vi "HFRR ADV v043.vi"() -> ()   [LabVIEW 2025] (continued)
      tunnel: [FALSE FALSE FALSE _ FALSE _ _ _ _ _ _ _ _ _ _ _ _ _ _ _ _ _ _ _ _ _ _ _ _ _ _ _ _ _ _ _ _ _ _ _ _ _ _ _ _ _ _ _ _ _ _ _ _ _ _ _ TRUE] -> w383
      event Timeout {
        n287 = event-data() -> ()  [unwired: 1 in, 3 out]
        n288 = disable-structure shown="Disabled" {
          frame Disabled {
            n289 = local read "Auto Start Test"() -> (w397:bool)
            n290 = local read "RUN"() -> (w398:bool)
            n291 = Or(x=w398, y=w397) -> (x .or. y?=w396:bool)
            n292 = case shown="True" w396 {
              frame False {
                w399 = TRUE ("PAUSE")
                n293 = call "ELAPSED TIMER VI - abort test.vi"("RESET"=w399, "PAUSE"=w399) -> ()  [unwired: 7 in, 3 out]
              }
              frame True {
                n294 = local read "Stroke 2"() -> (w404:dbl)
                n295 = local read "FF 3"() -> (w406:dbl)
                n296 = Equal?(x=w404, y=0.95 ("Stroke 2")) -> (x = y?=w401:bool)
                n297 = Equal?(x=w406, y=0.0 ("FF 3")) -> (x = y?=w402:bool)
                n298 = Or(x=w402, y=w401) -> (x .or. y?=w400:bool)
                n299 = case shown="True" w400 {
                  selector: w400 -> [_ w411]
                  frame False {
                    w407 = TRUE ("PAUSE")
                    n300 = call "ELAPSED TIMER VI - abort test.vi"("RESET"=w407, "PAUSE"=w407) -> ()  [unwired: 7 in, 3 out]
                  }
                  frame True {
                    n301 = Not(x=w411) -> (.not. x?=w410:bool)
                    n302 = call "ELAPSED TIMER VI - abort test.vi"("TARGET"=60.0, "RESET"=w410, "PAUSE"=FALSE) -> ("ELAPSED INDICATION"=w408:bool)  [unwired: 6 in, 2 out]
                    n303 = case shown="True" w408 {
                      frame False {
                      }
                      frame True {
                        n304 = stacked-sequence {
                          frame #0 {
                            w413 = FALSE
                            n305 = local write "RUN"(w413) -> ()
                            n306 = local write "Auto Start Test"(w413) -> ()
                          }
                          frame #1 {
                            n307 = One Button Dialog(message="Test stopped due to a communication error. Reconnect the C1 and C2 cables.") -> ()  [unwired: 1 in, 1 out]
                          }
                        }
                      }
                    }
                  }
                }
              }
            }
          }
          frame Enabled {
          }
        }
        n308 = Get Date/Time In Seconds() -> (seconds since 1Jan1904=w394:timestamp)
        n309 = Format Into String(format string="%<%I:%M:%S:%p %d:%B:%Y>T", w394) -> (resulting string=→"Time Stamp":string)  [unwired: 2 in, 1 out]
        n310 = local read "Service Password enable"() -> (w386:bool)
        n311 = local read "FILE"() -> (w391:string)
        n312 = call <vilib>:"Trim Whitespace.vi"("string"=w391) -> ("trimmed string"=w390:string)  [unwired: 1 in]
        n313 = String Length(string=w390) -> (length=w389:i32)
        n314 = Greater?(x=w389, y=1) -> (0:w387:bool)
        n315 = case shown="False" w387 {
          tunnel: w386 -> [w415 _]
          frame False {
            n316 = case shown="False" w415 {
              frame True {
                w416 = "Test Start In Service Mode" ("Tip Strip")
                w417 = T19."Enabled" ("Disabled")
                n317 = property on="Auto Start Test" class="Bool (strict)"("DisabledEnum"=w417, "TipStrip"=w416) -> ()  [unwired: 2 in, 2 out]
                n318 = property on="RUN" class="Bool (strict)"("DisabledEnum"=w417, "TipStrip"=w416) -> ()  [unwired: 2 in, 2 out]
              }
              frame False {
                w418 = "Enter File Name to Start Test" ("Tip Strip")
                w419 = T19."Disabled and Grayed Out" ("Disabled")
                n319 = property on="Auto Start Test" class="Bool (strict)"("DisabledEnum"=w419, "TipStrip"=w418) -> ()  [unwired: 2 in, 2 out]
                n320 = property on="RUN" class="Bool (strict)"("DisabledEnum"=w419, "TipStrip"=w418) -> ()  [unwired: 2 in, 2 out]
              }
            }
          }
          frame True {
            w420 = "" ("Tip Strip")
            w421 = T19."Enabled" ("Disabled")
            n321 = property on="Auto Start Test" class="Bool (strict)"("DisabledEnum"=w421, "TipStrip"=w420) -> ()  [unwired: 2 in, 2 out]
            n322 = property on="RUN" class="Bool (strict)"("DisabledEnum"=w421, "TipStrip"=w420) -> ()  [unwired: 2 in, 2 out]
          }
        }
      }
      event "RUN": Value Change {
        n323 = event-data() -> ()  [unwired: 1 in, 6 out]
        n324 = local read "RUN"() -> (w423:bool)
        n325 = case shown="False" w423 {
          frame False {
            n326 = flat-sequence {
              frame #0 {
                n327 = local write "START TEMP"(FALSE ("START TEMP")) -> ()
              }
              frame #1 {
                n328 = Wait (ms)(milliseconds to wait=u32 1500) -> ()  [unwired: 1 out]
              }
              frame #2 {
                n329 = local write "Humidity 2"(TRUE ("Humidity")) -> ()
              }
              frame #3 {
                n330 = local write "Due Write"("VC;0") -> ()
              }
              frame #4 {
                n331 = Wait (ms)(milliseconds to wait=u32 1500) -> ()  [unwired: 1 out]
              }
              frame #5 {
                w433 = T19."Enabled" ("Disabled")
                (unwired) T25."Imaging" ("Main Dashboard Buttons")
                (unwired) T21."Adv Scar" ("Main Tab")
                w435 = "" ("FILE")
                n332 = local write "measured_stroke"(0.0 ("measured_stroke")) -> ()
                n333 = local write "Due Write"("VC;0") -> ()
                n334 = local write "FILE"(w435) -> ()
                n335 = local write "Batch Ref Num :"(w435) -> ()
                n336 = local write "Fuel Discription :"(w435) -> ()
                n337 = local write "Main Tab"(T2."Adv Scar" ("Main Tab")) -> ()
                n338 = local write "Remarks :"(w435) -> ()
                n339 = local write "Main Dashboard Buttons"(T1."Imaging" ("Main Dashboard Buttons")) -> ()
                n340 = local write "TEST FILE NAM,E SAVED"(FALSE ("TEST FILE NAM,E SAVED")) -> ()
                n341 = property on="Stroke ( mm )" class="WFChart (strict)"("History Data"=cluster{"y":dbl, dbl, "y":dbl}[] []) -> ()  [unwired: 2 in, 2 out]
                n342 = property on="Auto Start Test" class="Bool (strict)"("Visible"=TRUE) -> ()  [unwired: 2 in, 2 out]
                n343 = property on="FRICVALZ 2" class="Bool (strict)"("DisabledEnum"=w433) -> ()  [unwired: 2 in, 2 out]
                n344 = property on="FRICVALZ 4" class="Bool (strict)"("DisabledEnum"=w433) -> ()  [unwired: 2 in, 2 out]
                n345 = property on="FRICVALZ 3" class="Bool (strict)"("DisabledEnum"=w433) -> ()  [unwired: 2 in, 2 out]
              }
            }
          }
          frame True {
            n346 = stacked-sequence {
              frame #0 {
                n347 = local write "FRICVALZ 4"(TRUE ("FRICVALZ 4")) -> ()
                n348 = local write "Due Write"("DAC;200") -> ()
              }
              frame #1 {
              }
              frame #2 {
              }
              frame #3 {
                n349 = Wait (ms)(milliseconds to wait=u32 1000) -> ()  [unwired: 1 out]
              }
              frame #4 {
                n350 = local write "Due Write"("VC;1") -> ()
              }
              frame #5 {
                n351 = Wait (ms)(milliseconds to wait=u32 1000) -> ()  [unwired: 1 out]
              }
              frame #6 {
                n352 = local write "Due Write"("VC;1") -> ()
              }
              frame #7 {
                n353 = Wait (ms)(milliseconds to wait=u32 1500) -> ()  [unwired: 1 out]
              }
              frame #8 {
                w446 = T19."Disabled" ("Disabled")
                n354 = property on="Auto Start Test" class="Bool (strict)"("Visible"=FALSE) -> ()  [unwired: 2 in, 2 out]
                n355 = local write "START TEMP"(TRUE ("START TEMP")) -> ()
                n356 = property on="FRICVALZ 2" class="Bool (strict)"("DisabledEnum"=w446) -> ()  [unwired: 2 in, 2 out]
                n357 = property on="FRICVALZ 4" class="Bool (strict)"("DisabledEnum"=w446) -> ()  [unwired: 2 in, 2 out]
                n358 = property on="FRICVALZ 3" class="Bool (strict)"("DisabledEnum"=w446) -> ()  [unwired: 2 in, 2 out]
              }
            }
          }
        }
      }
      event "run test Calibration": Value Change {
        n359 = event-data() -> ()  [unwired: 1 in, 6 out]
        n360 = local read "run test Calibration"() -> (w448:bool)
        n361 = case shown="False" w448 {
          frame False {
            n362 = flat-sequence {
              frame #0 {
                n363 = local write "START TEMP"(FALSE ("START TEMP")) -> ()
              }
              frame #1 {
                n364 = Wait (ms)(milliseconds to wait=u32 1500) -> ()  [unwired: 1 out]
              }
              frame #2 {
              }
              frame #3 {
                n365 = local write "Due Write"("VC;0") -> ()
              }
              frame #4 {
                n366 = Wait (ms)(milliseconds to wait=u32 1500) -> ()  [unwired: 1 out]
              }
              frame #5 {
                n367 = local write "Due Write"("VC;0") -> ()
                n368 = property on="Tab Control 6" class="TabCtl (strict)"("Visible"=FALSE) -> ()  [unwired: 2 in, 2 out]
                n369 = local write "Friction Force Calibration Result Tab"(enum32{"Calibration Results", "Page 2"}."Calibration Results" ("Friction Force Calibration Result Tab")) -> ()
                n370 = property on="Friction Force Calibration Result Tab" class="TabCtl (strict)"("Visible"=TRUE) -> ()  [unwired: 2 in, 2 out]
              }
            }
          }
          frame True {
            n371 = flat-sequence {
              frame #0 {
                n372 = local write "Due Write"("VC;1") -> ()
              }
              frame #1 {
                n373 = Wait (ms)(milliseconds to wait=u32 1000) -> ()  [unwired: 1 out]
              }
              frame #2 {
                n374 = local write "Due Write"("VC;1") -> ()
              }
              frame #3 {
                n375 = Wait (ms)(milliseconds to wait=u32 2000) -> ()  [unwired: 1 out]
              }
              frame #4 {
                n376 = local write "START TEMP"(TRUE ("START TEMP")) -> ()
                n377 = property on="Tab Control 6" class="TabCtl (strict)"("Visible"=TRUE) -> ()  [unwired: 2 in, 2 out]
                n378 = local write "Friction Force Calibration Result Tab"(enum32{"Calibration Results", "Page 2"}."Calibration Results" ("Friction Force Calibration Result Tab")) -> ()
              }
            }
          }
        }
      }
      event "Auto": Value Change {
        n379 = event-data() -> ()  [unwired: 1 in, 6 out]
        n380 = stacked-sequence {
          frame #0 {
            n381 = local write "FILE"("") -> ()
          }
          frame #1 {
            n382 = Get Date/Time In Seconds() -> (seconds since 1Jan1904=w469:timestamp)
            n383 = Format Into String(format string="%<%I_%M_%S_%p_%d_%B_%Y>T", w469) -> (resulting string=w468:string)  [unwired: 2 in, 1 out]
            n384 = local write "FILE"(w468) -> ()
          }
        }
        n385 = local read "Auto"() -> (w466:bool)
        n386 = Not(x=w466) -> (.not. x?=w465:bool)
        n387 = local write "Auto"(w465) -> ()
      }
      event "Auto Start Temp": Value Change {
        n388 = event-data() -> ()  [unwired: 1 in, 6 out]
        n389 = local read "Auto Start Test"() -> (w472:bool)
        n390 = case shown="False" w472 {
          frame False {
            n391 = stacked-sequence {
              frame #0 {
                n392 = local write "START TEMP"(FALSE ("START TEMP")) -> ()
              }
              frame #1 {
                n393 = Wait (ms)(milliseconds to wait=u32 2000) -> ()  [unwired: 1 out]
              }
              frame #2 {
                n394 = local write "Due Write"("VC;0") -> ()
              }
              frame #3 {
                n395 = Wait (ms)(milliseconds to wait=u32 2000) -> ()  [unwired: 1 out]
              }
              frame #4 {
                w483 = T19."Enabled" ("Disabled")
                (unwired) T25."Imaging" ("Main Dashboard Buttons")
                w484 = "" ("FILE")
                n396 = local write "Main Tab"(T2."Adv Scar" ("Main Tab")) -> ()
                n397 = local write "measured_stroke"(0.0 ("measured_stroke")) -> ()
                n398 = local write "Main Dashboard Buttons"(T1."Imaging" ("Main Dashboard Buttons")) -> ()
                n399 = property on="RUN" class="Bool (strict)"("Visible"=TRUE) -> ()  [unwired: 2 in, 2 out]
                n400 = local write "Due Write"("VC;0") -> ()
                n401 = local write "Humidity 2"(TRUE ("Humidity")) -> ()
                n402 = local write "TEST FILE NAM,E SAVED"(FALSE ("TEST FILE NAM,E SAVED")) -> ()
                n403 = local write "Fuel Discription :"(w484) -> ()
                n404 = local write "Batch Ref Num :"(w484) -> ()
                n405 = local write "Remarks :"(w484) -> ()
                n406 = local write "FILE"(w484) -> ()
                n407 = property on="FRICVALZ 2" class="Bool (strict)"("DisabledEnum"=w483) -> ()  [unwired: 2 in, 2 out]
                n408 = property on="FRICVALZ 4" class="Bool (strict)"("DisabledEnum"=w483) -> ()  [unwired: 2 in, 2 out]
                n409 = property on="FRICVALZ 3" class="Bool (strict)"("DisabledEnum"=w483) -> ()  [unwired: 2 in, 2 out]
              }
            }
          }
          frame True {
            n410 = stacked-sequence {
              frame #0 {
                n411 = local write "Due Write"("DAC;200") -> ()
              }
              frame #1 {
                n412 = Wait (ms)(milliseconds to wait=u32 1000) -> ()  [unwired: 1 out]
              }
              frame #2 {
              }
              frame #3 {
              }
              frame #4 {
                n413 = local write "Due Write"("VC;1") -> ()
              }
              frame #5 {
                n414 = Wait (ms)(milliseconds to wait=u32 1000) -> ()  [unwired: 1 out]
              }
              frame #6 {
                n415 = local write "Due Write"("VC;1") -> ()
              }
              frame #7 {
                n416 = Wait (ms)(milliseconds to wait=u32 1500) -> ()  [unwired: 1 out]
              }
              frame #8 {
                w493 = T19."Disabled" ("Disabled")
                n417 = property on="RUN" class="Bool (strict)"("Visible"=FALSE) -> ()  [unwired: 2 in, 2 out]
                n418 = property on="FRICVALZ 2" class="Bool (strict)"("DisabledEnum"=w493) -> ()  [unwired: 2 in, 2 out]
                n419 = property on="FRICVALZ 4" class="Bool (strict)"("DisabledEnum"=w493) -> ()  [unwired: 2 in, 2 out]
                n420 = property on="FRICVALZ 3" class="Bool (strict)"("DisabledEnum"=w493) -> ()  [unwired: 2 in, 2 out]
                "START TEMP" <- TRUE
              }
            }
          }
        }
      }
      event "FILE", "USERNAME", "USER ID": Mouse Enter {
        n421 = event-data() -> ()  [unwired: 1 in, 4 out]
        n422 = dll-call lib="kernel32.dll" fn="Wow64DisableWow64FsRedirection"("OldValue"=0) -> (error out=w500:errorcluster, "OldValue"=w498:i32)  [unwired: 4 in, 1 out]
        n423 = call <vilib>:"System Exec.vi"("run minimized? (F)"=TRUE, "error in (no error)"=w500, "command line"="C:\\Program Files\\Common Files\\Microsoft Shared\\Ink\\TabTip.exe") -> ("error out"=w499:errorcluster)  [unwired: 5 in, 3 out]
        n424 = dll-call lib="kernel32.dll" fn="Wow64EnableWow64FsRedirection"(error in=w499, "OldValue"=w498) -> ()  [unwired: 4 in, 2 out]
      }
      event "EDIT": Value Change {
        n425 = event-data() -> ()  [unwired: 1 in, 6 out]
        n426 = local read "EDIT"() -> (w501:bool)
        n427 = case shown="False" w501 {
          frame False {
            n428 = control-ref of="This VI"() -> (w518:refnum<vi>)
            n429 = property class="VI"(reference=w518) -> (reference out=w509:refnum<vi>, error out=w513:errorcluster, "Panel"=w517:refnum<vi>)  [unwired: 1 in]
            n430 = property class="Pnl"(reference=w517, error in=w513) -> (reference out=w511:refnum<vi>, error out=w514:errorcluster, "Panes[]"=w516:refnum<vi>[])
            n431 = for {
              tunnel: w516 -> [w524] mode=indexing
              tunnel: T24."Always Off" ("Horizontal Scrollbar Visibility") -> [w523]
              tunnel: w514 -> [w520]
              tunnel: [w519] -> w512
              n432 = property class="Pane"(reference=w524, error in=w520, "HorizScrollbarVisibility"=w523) -> (reference out=w521:refnum<vi>, error out=w522:errorcluster)
              n433 = Close Reference(reference=w521, error in (no error)=w522) -> (error out=w519:errorcluster)
            }
            n434 = Close Reference(reference=w511, error in (no error)=w512) -> (error out=w510:errorcluster)
            n435 = Close Reference(reference=w509, error in (no error)=w510) -> (error out=w504:errorcluster)
            "error out 7" <- w504
            n436 = call <vilib>:"Clear Errors.vi"("error in (no error)"=w504) -> ("error out"=w503:errorcluster)  [unwired: 5 in, 1 out]
            n437 = local write "Service Password enable"(FALSE ("Service Password enable")) -> ()
            n438 = call <userlib>:"Fit VI window to Largest Dec.vi"("error in (no error)"=w503, "border spacing (2 px)"=1) -> ("error out"=w508:errorcluster, "dup VI Ref"=w506:refnum<vi>)  [unwired: 4 in]
            n439 = invoke on="Invoke Node" class="VI" method="FP.Run-Time Position.Maximized"(reference=w506, error in=w508) -> (error out=w507:errorcluster)  [unwired: 2 in, 3 out]
            n440 = call <vilib>:"Clear Errors.vi"("error in (no error)"=w507) -> ()  [unwired: 5 in, 2 out]
          }
          frame True {
          }
        }
      }
      event "Heater Button": Value Change {
        n441 = event-data() -> ()  [unwired: 1 in, 6 out]
        n442 = local read "Heater Button"() -> (w525:bool)
        n443 = case shown="True" w525 {
          frame True {
            n444 = stacked-sequence {
              frame #0 {
                n445 = Wait (ms)(milliseconds to wait=u32 1500) -> ()  [unwired: 1 out]
              }
              frame #1 {
                n446 = local read "Set Temp"() -> (w527:dbl)
                n447 = Number To Fractional String(number=w527, precision (6)=i16 2) -> (F-format string=w530:string)  [unwired: 2 in]
                n448 = Concatenate Strings("ST;" ("Command"), w530) -> (w529:string)
                n449 = local write "Due Write"(w529) -> ()
              }
              frame #2 {
                n450 = Wait (ms)(milliseconds to wait=u32 1500) -> ()  [unwired: 1 out]
              }
              frame #3 {
                n451 = local write "Due Write"("HE;1" ("Command")) -> ()
              }
              frame #4 {
                n452 = Wait (ms)(milliseconds to wait=u32 1500) -> ()  [unwired: 1 out]
              }
              frame #5 {
                n453 = stacked-sequence {
                  frame #0 {
                    n454 = Wait (ms)(milliseconds to wait=u32 1500) -> ()  [unwired: 1 out]
                  }
                  frame #1 {
                    n455 = local read "Set Temp"() -> (w536:dbl)
                    n456 = Number To Fractional String(number=w536, precision (6)=i16 2) -> (F-format string=w539:string)  [unwired: 2 in]
                    n457 = Concatenate Strings("ST;" ("Command"), w539) -> (w538:string)
                    n458 = local write "Due Write"(w538) -> ()
                  }
                  frame #2 {
                    n459 = Wait (ms)(milliseconds to wait=u32 1500) -> ()  [unwired: 1 out]
                  }
                  frame #3 {
                    n460 = local write "Due Write"("HE;1" ("Command")) -> ()
                  }
                  frame #4 {
                    n461 = Wait (ms)(milliseconds to wait=u32 1500) -> ()  [unwired: 1 out]
                  }
                }
              }
            }
          }
          frame False {
            n462 = stacked-sequence {
              frame #0 {
                n463 = Wait (ms)(milliseconds to wait=u32 1500) -> ()  [unwired: 1 out]
              }
              frame #1 {
                n464 = Concatenate Strings("ST;" ("Command"), "0" ("string")) -> (w546:string)
                n465 = local write "Due Write"(w546) -> ()
              }
              frame #2 {
                n466 = Wait (ms)(milliseconds to wait=u32 1500) -> ()  [unwired: 1 out]
              }
              frame #3 {
                n467 = local write "Due Write"("HE;0" ("Command")) -> ()
              }
              frame #4 {
                n468 = Wait (ms)(milliseconds to wait=u32 1500) -> ()  [unwired: 1 out]
              }
            }
          }
        }
      }
      event "Headen Service Button": Value Change {
        n469 = event-data() -> ()  [unwired: 1 in, 6 out]
        n470 = local read "Headen Service Button"() -> (w551:bool)
        n471 = case shown="True" w551 {
          frame False {
            n472 = property on="Password 3" class="Clust (strict)"("Visible"=FALSE) -> ()  [unwired: 2 in, 2 out]
            n473 = property on="Service Password Log" class="Str"("Visible"=FALSE) -> ()  [unwired: 2 in, 2 out]
          }
          frame True {
            n474 = property on="Password 3" class="Clust (strict)"("Visible"=TRUE) -> ()  [unwired: 2 in, 2 out]
            n475 = property on="Service Password Log" class="Str"("Visible"=TRUE) -> ()  [unwired: 2 in, 2 out]
          }
        }
      }
      event "Password 3.Service Password": Value Change {
        n476 = event-data() -> ()  [unwired: 1 in, 6 out]
        n477 = Unbundle By Name("Password 3") -> ("Service Password"=w558:string)
        n478 = call <vilib>:"Trim Whitespace.vi"("string"=w558) -> ("trimmed string"=w556:string)  [unwired: 1 in]
        n479 = Equal?(x=w556, y="Service@123") -> (x = y?=w557:bool)
        n480 = case shown="False" w557 {
          selector: w557 -> [w561 w563]
          frame False {
            n481 = local write "Service Password enable"(w561) -> ()
            n482 = property on="Service Password Log" class="Str"("Visible"=TRUE) -> ()  [unwired: 2 in, 2 out]
          }
          frame True {
            n483 = property on="Service Password Log" class="Str"("Visible"=FALSE) -> ()  [unwired: 2 in, 2 out]
            "Service Password enable" <- w563
          }
        }
      }
      event "Sign In": Value Change {
        w565 = FALSE ("Visible")
        n484 = event-data() -> ()  [unwired: 1 in, 6 out]
        n485 = property on="About" class="Clust (strict)"("Visible"=w565) -> ()  [unwired: 2 in, 2 out]
        n486 = property on="Password 3" class="Clust (strict)"("Visible"=w565) -> ()  [unwired: 2 in, 2 out]
        n487 = property on="Service Password Log" class="Str"("Visible"=FALSE) -> ()  [unwired: 2 in, 2 out]
      }
      event "Info": Value Change {
        n488 = event-data() -> ()  [unwired: 1 in, 6 out]
        n489 = local read "Info"() -> (w567:bool)
        n490 = case shown="False" w567 {
          frame False {
            n491 = property on="About" class="Clust (strict)"("Visible"=FALSE) -> ()  [unwired: 2 in, 2 out]
          }
          frame True {
            n492 = property on="About" class="Clust (strict)"("Visible"=TRUE) -> ()  [unwired: 2 in, 2 out]
          }
        }
      }
      event "Calibration": Value Change {
        n493 = event-data() -> ()  [unwired: 1 in, 6 out]
        n494 = local read "Calibration"() -> (w571:bool)
        n495 = case shown="False" w571 {
          frame False {
            n496 = property on="Calibration 2" class="TabCtl (strict)"("Visible"=FALSE) -> ()  [unwired: 2 in, 2 out]
            n497 = local write "Cal Password"("" ("Cal Password")) -> ()
          }
          frame True {
            n498 = property on="Calibration 2" class="TabCtl (strict)"("Visible"=TRUE) -> ()  [unwired: 2 in, 2 out]
            n499 = local write "Cal Password"("" ("Cal Password")) -> ()
          }
        }
        n500 = property on="Wrong Password" class="Str"("Visible"=FALSE) -> ()  [unwired: 2 in, 2 out]
      }
      event "Cal Password": Value Change {
        n501 = event-data() -> ()  [unwired: 1 in, 6 out]
        n502 = local read "Cal Password"() -> (w579:string)
        n503 = call <vilib>:"Trim Whitespace.vi"("string"=w579) -> ("trimmed string"=w578:string)  [unwired: 1 in]
        n504 = Equal?(x=w578, y="Cal@321") -> (x = y?=w576:bool)
        n505 = case shown="True" w576 {
          frame False {
            n506 = property on="Wrong Password" class="Str"("Visible"=TRUE) -> ()  [unwired: 2 in, 2 out]
          }
          frame True {
            n507 = property on="Wrong Password" class="Str"("Visible"=FALSE) -> ()  [unwired: 2 in, 2 out]
            n508 = local write "Main Tab"(T2."About" ("Main Tab")) -> ()
            n509 = local write "Cal Password"("" ("Cal Password")) -> ()
            n510 = local write "Main Dashboard Buttons"(T1."About" ("Main Dashboard Buttons")) -> ()
            n511 = property on="Calibration 2" class="TabCtl (strict)"("Visible"=FALSE) -> ()  [unwired: 2 in, 2 out]
            n512 = local write "Calibration"(FALSE ("Calibration")) -> ()
          }
        }
      }
      event "Calibration Selection": Value Change {
        n513 = event-data() -> ()  [unwired: 1 in, 6 out]
        n514 = local read "Calibration Selection"() -> (w588:T8)
        n515 = case shown="\"Stroke Calibration\"" w588 {
          tunnel: [T7."Stroke" ("Main Calibration Tab") T7."Friction" ("Main Calibration Tab") T7."Main" ("Main Calibration Tab") T7."Temperature" ("Main Calibration Tab")] -> w587
          frame "Stroke Calibration" {
          }
          frame "Friction Force Calibration" {
          }
          frame Default {
          }
          frame "Temperature Calibration" {
          }
        }
        n516 = local write "Main Calibration Tab"(w587) -> ()
      }
      event "Back Stroke": Value Change {
        n517 = event-data() -> ()  [unwired: 1 in, 6 out]
        n518 = local write "Main Stroke Tab"(T9."Step 1" ("Main Stroke Tab")) -> ()
        n519 = local write "Main Calibration Tab"(T7."Main" ("Main Calibration Tab")) -> ()
        n520 = local write "Back Stroke"(FALSE ("Back Stroke")) -> ()
        n521 = local write "Calibration Selection"(T8."Default" ("Calibration Selection")) -> ()
      }
      event "Step 2 Back": Value Change {
        n522 = event-data() -> ()  [unwired: 1 in, 6 out]
        n523 = local write "Main Stroke Tab"(T9."Step 1" ("Main Stroke Tab")) -> ()
        n524 = local write "Step 2 Back"(FALSE ("Back Stroke")) -> ()
        n525 = local write "Calibration Selection"(T8."Default" ("Calibration Selection")) -> ()
      }
      event "Step 3 Back": Value Change {
        n526 = event-data() -> ()  [unwired: 1 in, 6 out]
        n527 = local write "Main Stroke Tab"(T9."Step 2" ("Main Stroke Tab")) -> ()
        n528 = local write "Step 3 Back"(FALSE ("Back Stroke")) -> ()
        n529 = local write "Calibration Selection"(T8."Default" ("Calibration Selection")) -> ()
      }
      event "Step 4 Back": Value Change {
        n530 = event-data() -> ()  [unwired: 1 in, 6 out]
        n531 = local write "Main Stroke Tab"(T9."Step 3" ("Main Stroke Tab")) -> ()
        n532 = local write "Step 4 Back"(FALSE ("Back Stroke")) -> ()
        n533 = local write "Calibration Selection"(T8."Default" ("Calibration Selection")) -> ()
      }
      event "Step 5 Back": Value Change {
        n534 = event-data() -> ()  [unwired: 1 in, 6 out]
        n535 = local write "Main Stroke Tab"(T9."Step 4" ("Main Stroke Tab")) -> ()
        n536 = local write "Step 5 Back"(FALSE ("Back Stroke")) -> ()
        n537 = local write "Calibration Selection"(T8."Default" ("Calibration Selection")) -> ()
      }
      event "Step 6 Back": Value Change {
        n538 = event-data() -> ()  [unwired: 1 in, 6 out]
        n539 = local write "Main Stroke Tab"(T9."Step 5" ("Main Stroke Tab")) -> ()
        n540 = local write "Step 6 Back"(FALSE ("Back Stroke")) -> ()
        n541 = local write "Calibration Selection"(T8."Default" ("Calibration Selection")) -> ()
      }
      event "Back Stroke step 7": Value Change {
        n542 = event-data() -> ()  [unwired: 1 in, 6 out]
        n543 = local write "Main Stroke Tab"(T9."Step 5" ("Main Stroke Tab")) -> ()
        n544 = local write "Back Stroke step 7"(FALSE ("Back Stroke")) -> ()
        n545 = local write "Calibration Selection"(T8."Default" ("Calibration Selection")) -> ()
      }
      event "Back Stroke step 8": Value Change {
        n546 = event-data() -> ()  [unwired: 1 in, 6 out]
        n547 = local write "Main Stroke Tab"(T9."Step 7" ("Main Stroke Tab")) -> ()
        n548 = local write "Back Stroke step 8"(FALSE ("Back Stroke")) -> ()
        n549 = local write "Calibration Selection"(T8."Default" ("Calibration Selection")) -> ()
      }
      event "Back Stroke 8": Value Change {
        n550 = event-data() -> ()  [unwired: 1 in, 6 out]
        n551 = local write "MOVE CARRIAGE TO"(1.0 ("MOVE CARRIAGE TO")) -> ()
        n552 = local write "Main Stroke Tab"(T9."Step 1" ("Main Stroke Tab")) -> ()
        n553 = local write "Calibration Selection"(T8."Default" ("Calibration Selection")) -> ()
        n554 = local write "Back Stroke 8"(FALSE ("Back Stroke 8")) -> ()
      }
      event "Continue Stroke": Value Change {
        n555 = event-data() -> ()  [unwired: 1 in, 6 out]
        n556 = local write "Main Stroke Tab"(T9."Step 2" ("Main Stroke Tab")) -> ()
        n557 = local write "Continue Stroke"(FALSE ("Continue Stroke")) -> ()
      }
      event "Continue Stroke step 2": Value Change {
        n558 = event-data() -> ()  [unwired: 1 in, 6 out]
        n559 = local write "Main Stroke Tab"(T9."Step 3" ("Main Stroke Tab")) -> ()
        n560 = local write "Continue Stroke step 2"(FALSE ("Continue Stroke")) -> ()
      }
      event "Continue Stroke step 3": Value Change {
        n561 = event-data() -> ()  [unwired: 1 in, 6 out]
        n562 = local write "Main Stroke Tab"(T9."Step 4" ("Main Stroke Tab")) -> ()
        n563 = local write "Continue Stroke step 3"(FALSE ("Continue Stroke")) -> ()
      }
      event "Continue Stroke step 4": Value Change {
        n564 = event-data() -> ()  [unwired: 1 in, 6 out]
        n565 = local write "Main Stroke Tab"(T9."Step 5" ("Main Stroke Tab")) -> ()
        n566 = local write "Continue Stroke step 4"(FALSE ("Continue Stroke")) -> ()
      }
      event "Continue Stroke step 5": Value Change {
        n567 = event-data() -> ()  [unwired: 1 in, 6 out]
        n568 = local write "Main Stroke Tab"(T9."Step 7" ("Main Stroke Tab")) -> ()
        n569 = local write "Continue Stroke step 5"(FALSE ("Continue Stroke")) -> ()
      }
      event "Continue Stroke step 6": Value Change {
        n570 = event-data() -> ()  [unwired: 1 in, 6 out]
        n571 = local write "Main Stroke Tab"(T9."Step 7" ("Main Stroke Tab")) -> ()
        n572 = local write "Continue Stroke step 6"(FALSE ("Continue Stroke")) -> ()
      }
      event "Continue Stroke step 7": Value Change {
        w636 = FALSE ("0.2mm")
        n573 = event-data() -> ()  [unwired: 1 in, 6 out]
        n574 = local write "0.4 mm"(w636) -> ()
        n575 = local write "0.6 mm"(w636) -> ()
        n576 = local write "1.0 mm"(w636) -> ()
        n577 = local write "1.2 mm"(w636) -> ()
        n578 = local write "0.2 2"(w636) -> ()
        n579 = local write "0.4 2"(w636) -> ()
        n580 = local write "0.6 2"(w636) -> ()
        n581 = local write "0.8 2"(w636) -> ()
        n582 = local write "1.0 2"(w636) -> ()
        n583 = local write "1.2"(w636) -> ()
        n584 = local write "0.2mm"(w636) -> ()
        n585 = local write "0.8mm"(w636) -> ()
        n586 = local write "Main Stroke Tab"(T9."Step 8" ("Main Stroke Tab")) -> ()
        n587 = local write "Continue Stroke step 7"(FALSE ("Continue Stroke")) -> ()
        n588 = local write "Stroke Test Complete"(T10."Test Progress" ("Stroke Test Complete")) -> ()
        "Position Measurment Temp" <- 4.0 ("Position Measurment Temp")
        "Calibration Tare" <- TRUE ("Calibration Tare")
        "MOVE CARRIAGE TO" <- 1.0 ("MOVE CARRIAGE TO")
      }
      event "Continue Stroke step 8": Value Change {
        n589 = event-data() -> ()  [unwired: 1 in, 6 out]
        n590 = local read "LVDT STROKE  Calibration"() -> (w641:dbl)
        n591 = local read "Position Measurment Temp"() -> (w642:dbl)
        n592 = case shown="7" w642 {
          selector: w642 -> [w647 w652 w657 w662 _ w670 w673 w674]
          tunnel: w641 -> [w643 w648 w653 w658 w664 w667 _ _]
          frame 0, Default {
            w645 = TRUE ("0.2mm")
            n593 = Increment(x=w647) -> (x+1=w646:i32)
            n594 = local write "Position Measurment Temp"(w646) -> ()
            n595 = local write "0.2mm"(w645) -> ()
            n596 = local write "0.2 2"(w645) -> ()
            n597 = local write "MOVE CARRIAGE TO"(1.0 ("MOVE CARRIAGE TO")) -> ()
            "Calibration 0.2" <- w643
          }
          frame 1 {
            w650 = TRUE ("0.4 mm")
            n598 = Increment(x=w652) -> (x+1=w651:i32)
            n599 = local write "Calibration 0.4"(w648) -> ()
            n600 = local write "Position Measurment Temp"(w651) -> ()
            n601 = local write "0.4 mm"(w650) -> ()
            n602 = local write "MOVE CARRIAGE TO"(0.6 ("MOVE CARRIAGE TO")) -> ()
            n603 = local write "0.4 2"(w650) -> ()
          }
          frame 2 {
            w655 = TRUE ("0.6 mm")
            n604 = Increment(x=w657) -> (x+1=w656:i32)
            n605 = local write "Calibration 0.6"(w653) -> ()
            n606 = local write "Position Measurment Temp"(w656) -> ()
            n607 = local write "0.6 2"(w655) -> ()
            n608 = local write "0.6 mm"(w655) -> ()
            n609 = local write "MOVE CARRIAGE TO"(0.8 ("MOVE CARRIAGE TO")) -> ()
          }
          frame 3 {
            w659 = TRUE ("0.6 mm")
            n610 = Increment(x=w662) -> (x+1=w661:i32)
            n611 = local write "Position Measurment Temp"(w661) -> ()
            n612 = local write "MOVE CARRIAGE TO"(1.0 ("MOVE CARRIAGE TO")) -> ()
            n613 = local write "0.8mm"(w659) -> ()
            n614 = local write "0.8 2"(w659) -> ()
            "Calibration 0.8" <- w658
          }
          frame 4 {
            w665 = TRUE ("0.6 mm")
            n615 = local write "Position Measurment Temp"(6.0 ("Position Measurment Temp")) -> ()
            n616 = local write "MOVE CARRIAGE TO"(1.0 ("MOVE CARRIAGE TO")) -> ()
            n617 = local write "1.0 mm"(w665) -> ()
            n618 = local write "1.0 2"(w665) -> ()
            "Calibration 1.0" <- w664
          }
          frame 5 {
            w668 = TRUE ("0.6 mm")
            n619 = Increment(x=w670) -> (x+1=w669:i32)
            n620 = local write "Position Measurment Temp"(w669) -> ()
            n621 = local write "1.2 mm"(w668) -> ()
            n622 = local write "1.2"(w668) -> ()
            "Calibration 1.2" <- w667
          }
          frame 6 {
            n623 = Increment(x=w673) -> (x+1=w672:i32)
            n624 = local write "Position Measurment Temp"(w672) -> ()
            n625 = local write "Stroke Test Complete"(T10."Stroke Points Completed" ("Stroke Test Complete")) -> ()
          }
          frame 7 {
            n626 = stacked-sequence {
              tunnel: w674 -> [w675 _ _]
              frame #0 {
                n627 = Increment(x=w675) -> (x+1=w676:i32)
                n628 = local write "Main Stroke Tab"(T9."Step 9" ("Main Stroke Tab")) -> ()
                n629 = local write "Position Measurment Temp"(w676) -> ()
                n630 = Insert Into Array(array=dbl[] [], new element #1=0.2 ("new element/subarray"), new element #2=0.4 ("new element/subarray"), new element #3=0.6 ("new element/subarray"), new element #4=0.8 ("new element/subarray"), new element #5=1.0 ("new element/subarray"), new element #6=1.2 ("new element/subarray")) -> (→"1D stroke":dbl[])  [unwired: 1 in]
                n631 = local read "Calibration 0.2"() -> (w683:dbl)
                n632 = local read "Calibration 0.4"() -> (w682:dbl)
                n633 = local read "Calibration 0.6"() -> (w681:dbl)
                n634 = local read "Calibration 0.8"() -> (w680:dbl)
                n635 = local read "Calibration 1.0"() -> (w679:dbl)
                n636 = local read "Calibration 1.2"() -> (w678:dbl)
                n637 = Insert Into Array(array=dbl[] [], new element #1=w683, new element #2=w682, new element #3=w681, new element #4=w680, new element #5=w679, new element #6=w678) -> (→"Calibrated Voltage Value":dbl[])  [unwired: 1 in]
              }
              frame #1 {
                n638 = local read "calibration values"() -> (w706:dbl[])
                n639 = local read "Calibrated Voltage Value"() -> (w708:dbl[])
                n640 = Index Array(array=w706, index #1=1 ("index"), index #2=3 ("index"), index #3=5 ("index"), index #4=7 ("index"), index #5=9 ("index"), index #6=11 ("index")) -> (element #1=w699:dbl, element #2=w698:dbl, element #3=w697:dbl, element #4=w696:dbl, element #5=w695:dbl, element #6=w694:dbl)
                n641 = local read "1D stroke"() -> (w709:dbl[])
                n642 = for {
                  tunnel: [w718] -> w707 mode=indexing
                  tunnel: w709 -> [w717] mode=indexing
                  tunnel: w708 -> [w716] mode=indexing
                  tunnel: w699 -> [w715]
                  tunnel: w698 -> [w714]
                  tunnel: w697 -> [w713]
                  tunnel: w696 -> [w712]
                  tunnel: w695 -> [w711]
                  tunnel: w694 -> [w710]
                  n643 = formula code="if (stroke == 0.2)\n{\n    if ((voltage >= REF_02 - 0.2) && (voltage <= REF_02 + 0.2))\n        status = 1;\n    else\n        status = 0;\n}\nelse if (stroke == 0.4)\n{\n    if ((voltage >= REF_04 - 0.2) && (voltage <= REF_04 + 0.2))\n        status = 1;\n    else\n        status = 0;\n}\nelse if (stroke == 0.6)\n{\n    if ((voltage >= REF_06 - 0.2) && (voltage <= REF_06 + 0.2))\n        status = 1;\n    else\n        status = 0;\n}\nelse if (stroke == 0.8)\n{\n    if ((voltage >= REF_08 - 0.2) && (voltage <= REF_08 + 0.2))\n        status = 1;\n    else\n        status = 0;\n}\nelse if (stroke == 1.0)\n{\n    if ((voltage >= REF_10 - 1) && (voltage <= REF_10 + 1))\n        status = 1;\n    else\n        status = 0;\n}\nelse if (stroke == 1.2)\n{\n    if ((voltage >= REF_12 - 0.2) && (voltage <= REF_12 + 0.2))\n        status = 1;\n    else\n        status = 0;\n}\nelse\n{\n    status = 0;\n}"("stroke"=w717, "voltage"=w716, "REF_02"=w715, "REF_04"=w714, "REF_06"=w713, "REF_08"=w712, "REF_10"=w711, "REF_12"=w710) -> ("status"=w718:dbl)
                }
                "Status" <- w707
              }
              frame #2 {
                w725 = 1.0
                n644 = local read "Status"() -> (w732:dbl[])
                n645 = Index Array(array=w732) -> (element #1=w731:dbl, element #2=w730:dbl, element #3=w729:dbl, element #4=w728:dbl, element #5=w727:dbl, element #6=w726:dbl)  [unwired: 6 in]
                n646 = Equal?(x=w730, y=w725) -> (x = y?=w723:bool)
                n647 = Equal?(x=w729, y=w725) -> (x = y?=w722:bool)
                n648 = Equal?(x=w728, y=w725) -> (x = y?=w721:bool)
                n649 = Equal?(x=w727, y=w725) -> (x = y?=w720:bool)
                n650 = Equal?(x=w726, y=w725) -> (x = y?=w719:bool)
                n651 = Equal?(x=w731, y=w725) -> (x = y?=w724:bool)
                n652 = case shown="True" w724 {
                  selector: w724 -> [w743 w744]
                  frame True {
                    n653 = local write "Point 1 - 0.2 mm"(w743) -> ()
                    n654 = property on="Point 1 - 0.2 mm" class="Bool"("Caption.Visible"=w743) -> ()  [unwired: 2 in, 2 out]
                  }
                  frame False {
                    n655 = local write "Point 1 - 0.2 mm"(w744) -> ()
                    n656 = property on="Point 1 - 0.2 mm" class="Bool"("Caption.Visible"=w744) -> ()  [unwired: 2 in, 2 out]
                  }
                }
                n657 = case shown="True" w723 {
                  selector: w723 -> [w741 w742]
                  frame True {
                    n658 = local write "Point 2 - 0.4 mm"(w741) -> ()
                    n659 = property on="Point 2 - 0.4 mm" class="Bool"("Caption.Visible"=w741) -> ()  [unwired: 2 in, 2 out]
                  }
                  frame False {
                    n660 = local write "Point 2 - 0.4 mm"(w742) -> ()
                    n661 = property on="Point 2 - 0.4 mm" class="Bool"("Caption.Visible"=w742) -> ()  [unwired: 2 in, 2 out]
                  }
                }
                n662 = case shown="True" w720 {
                  selector: w720 -> [w735 w736]
                  frame True {
                    n663 = local write "Point 5 - 1.0 mm"(w735) -> ()
                    n664 = property on="Point 5 - 1.0 mm" class="Bool"("Caption.Visible"=w735) -> ()  [unwired: 2 in, 2 out]
                  }
                  frame False {
                    n665 = local write "Point 5 - 1.0 mm"(w736) -> ()
                    n666 = property on="Point 5 - 1.0 mm" class="Bool"("Caption.Visible"=w736) -> ()  [unwired: 2 in, 2 out]
                  }
                }
                n667 = case shown="True" w722 {
                  selector: w722 -> [w739 w740]
                  frame True {
                    n668 = local write "Point 3 - 0.6 mm"(w739) -> ()
                    n669 = property on="Point 3 - 0.6 mm" class="Bool"("Caption.Visible"=w739) -> ()  [unwired: 2 in, 2 out]
                  }
                  frame False {
                    n670 = local write "Point 3 - 0.6 mm"(w740) -> ()
                    n671 = property on="Point 3 - 0.6 mm" class="Bool"("Caption.Visible"=w740) -> ()  [unwired: 2 in, 2 out]
                  }
                }
                n672 = case shown="True" w721 {
                  selector: w721 -> [w737 w738]
                  frame True {
                    n673 = local write "Point 4 - 0.8 mm"(w737) -> ()
                    n674 = property on="Point 4 - 0.8 mm" class="Bool"("Caption.Visible"=w737) -> ()  [unwired: 2 in, 2 out]
                  }
                  frame False {
                    n675 = local write "Point 4 - 0.8 mm"(w738) -> ()
                    n676 = property on="Point 4 - 0.8 mm" class="Bool"("Caption.Visible"=w738) -> ()  [unwired: 2 in, 2 out]
                  }
                }
                n677 = case shown="True" w719 {
                  selector: w719 -> [w733 w734]
                  frame True {
                    n678 = local write "Point 6 - 1.2 mm"(w733) -> ()
                    n679 = property on="Point 6 - 1.2 mm" class="Bool"("Caption.Visible"=w733) -> ()  [unwired: 2 in, 2 out]
                  }
                  frame False {
                    n680 = local write "Point 6 - 1.2 mm"(w734) -> ()
                    n681 = property on="Point 6 - 1.2 mm" class="Bool"("Caption.Visible"=w734) -> ()  [unwired: 2 in, 2 out]
                  }
                }
              }
            }
          }
        }
      }
      event "Accept & Save": Value Change {
        n682 = event-data() -> ()  [unwired: 1 in, 6 out]
        n683 = flat-sequence {
          frame #0 {
            n684 = Get Date/Time In Seconds() -> (seconds since 1Jan1904=w747:timestamp)
            n685 = Format Into String(format string="%<%I:%M:%S:%p %d:%B:%Y>T", w747) -> (resulting string=w745:string)  [unwired: 2 in, 1 out]
            n686 = local write "STROKE CALIBRATION"(w745) -> ()
          }
          frame #1 {
            n687 = local write "Save Button"(TRUE ("Save Button")) -> ()
          }
          frame #2 {
            n688 = local write "MOVE CARRIAGE TO"(1.0 ("MOVE CARRIAGE TO")) -> ()
            n689 = local write "Main Calibration Tab"(T7."Main" ("Main Calibration Tab")) -> ()
            n690 = local write "Main Stroke Tab"(T9."Step 1" ("Main Stroke Tab")) -> ()
            n691 = local write "Calibration Selection"(T8."Default" ("Calibration Selection")) -> ()
            n692 = local write "Back Stroke 8"(FALSE ("Back Stroke 8")) -> ()
          }
        }
      }
      event "TEMPERATURE STEP Back 1", "TEMPERATURE STEP Back air Temp": Value Change {
        n693 = event-data() -> ()  [unwired: 1 in, 6 out]
        n694 = stacked-sequence {
          frame #0 {
            n695 = local write "Main Calibration Tab"(T7."Main" ("Main Calibration Tab")) -> ()
            n696 = local write "Tab Control 4"(T12."Main" ("Tab Control 4")) -> ()
            n697 = local write "Temperature Selection"(T13."Default" ("Temperature Selection")) -> ()
          }
          frame #1 {
            n698 = Wait (ms)(milliseconds to wait=u32 1000) -> ()  [unwired: 1 out]
            n699 = local write "Calibration Selection"(T8."Default" ("Calibration Selection")) -> ()
          }
          frame #2 {
            n700 = local write "Due Write"("CAL;END" ("Command")) -> ()
          }
          frame #3 {
            n701 = Wait (ms)(milliseconds to wait=u32 2000) -> ()  [unwired: 1 out]
          }
          frame #4 {
            n702 = local write "Due Write"("CAL;END" ("Command")) -> ()
          }
        }
      }
      event "Temperature Continue Step 1": Value Change {
        n703 = event-data() -> ()  [unwired: 1 in, 6 out]
        n704 = stacked-sequence {
          frame #0 {
            n705 = Wait (ms)(milliseconds to wait=u32 1000) -> ()  [unwired: 1 out]
          }
          frame #1 {
            n706 = local write "Due Write"("CAL;START" ("Command")) -> ()
          }
          frame #2 {
            n707 = Wait (ms)(milliseconds to wait=u32 500) -> ()  [unwired: 1 out]
          }
          frame #3 {
            n708 = local write "Due Write"("CAL;START" ("Command")) -> ()
          }
          frame #4 {
            n709 = Wait (ms)(milliseconds to wait=u32 1000) -> ()  [unwired: 1 out]
          }
          frame #5 {
          }
          frame #6 {
          }
          frame #7 {
          }
          frame #8 {
            n710 = local write "Tab Control 4"(T12."Step 2" ("Tab Control 4")) -> ()
          }
        }
      }
      event "Temperature Continue Step air Step 1": Value Change {
        n711 = event-data() -> ()  [unwired: 1 in, 6 out]
        n712 = stacked-sequence {
          frame #0 {
            n713 = Wait (ms)(milliseconds to wait=u32 1000) -> ()  [unwired: 1 out]
          }
          frame #1 {
            n714 = local write "Due Write"("CAL;START" ("Command")) -> ()
          }
          frame #2 {
            n715 = Wait (ms)(milliseconds to wait=u32 1000) -> ()  [unwired: 1 out]
          }
          frame #3 {
            n716 = local write "Due Write"("CAL;START" ("Command")) -> ()
          }
          frame #4 {
          }
          frame #5 {
          }
          frame #6 {
          }
          frame #7 {
          }
          frame #8 {
            n717 = local write "Tab Control 4"(T12."Air Step 2" ("Tab Control 4")) -> ()
          }
        }
      }
      event "Temperature Selection": Value Change {
        n718 = event-data() -> ()  [unwired: 1 in, 6 out]
        n719 = local read "Temperature Selection"() -> (w773:T13)
        n720 = case shown="\"Sample Temperature\"" w773 {
          frame "Air Temperature" {
            n721 = local write "Tab Control 4"(T12."Air Step 1" ("Tab Control 4")) -> ()
          }
          frame "Sample Temperature" {
            n722 = local write "Tab Control 4"(T12."Step 1" ("Tab Control 4")) -> ()
          }
          frame "Default", Default {
          }
        }
      }
      event "Temperature Continue Step 2": Value Change {
        n723 = event-data() -> ()  [unwired: 1 in, 6 out]
        n724 = stacked-sequence {
          frame #0 {
            n725 = stacked-sequence {
              frame #0 {
                n726 = Wait (ms)(milliseconds to wait=u32 1500) -> ()  [unwired: 1 out]
              }
              frame #1 {
                # "CAL;A1;<true_T>"
                n727 = local read "Sensor value"() -> (→"Sample 0deg temp":dbl)
                n728 = local write "Due Write"("CAL;A1;0" ("Command")) -> ()
              }
              frame #2 {
                n729 = Wait (ms)(milliseconds to wait=u32 1500) -> ()  [unwired: 1 out]
              }
              frame #3 {
                # "CAL;A1;<true_T>"
                n730 = local write "Due Write"("CAL;A1;0" ("Command")) -> ()
              }
              frame #4 {
              }
            }
          }
          frame #1 {
            n731 = local write "Tab Control 4"(T12."Step 3" ("Tab Control 4")) -> ()
          }
        }
      }
      event "Temperature Continue Air Step 2": Value Change {
        n732 = event-data() -> ()  [unwired: 1 in, 6 out]
        n733 = stacked-sequence {
          frame #0 {
            n734 = stacked-sequence {
              frame #0 {
                n735 = Wait (ms)(milliseconds to wait=u32 1000) -> ()  [unwired: 1 out]
              }
              frame #1 {
                # "CAL;A1;<true_T>"
                n736 = local write "Due Write"("CAL;A1;0" ("Command")) -> ()
              }
              frame #2 {
                n737 = Wait (ms)(milliseconds to wait=u32 1000) -> ()  [unwired: 1 out]
              }
              frame #3 {
                # "CAL;A1;<true_T>"
                n738 = local write "Due Write"("CAL;A1;0" ("Command")) -> ()
              }
              frame #4 {
                n739 = local read "Sensor value"() -> (→"Air 0deg temp":dbl)
              }
            }
          }
          frame #1 {
            n740 = local write "Tab Control 4"(T12."Air Step 3" ("Tab Control 4")) -> ()
          }
        }
      }
      event "Temperature Continue Step 3": Value Change {
        n741 = event-data() -> ()  [unwired: 1 in, 6 out]
        n742 = stacked-sequence {
          frame #0 {
            n743 = stacked-sequence {
              frame #0 {
                n744 = Wait (ms)(milliseconds to wait=u32 1500) -> ()  [unwired: 1 out]
              }
              frame #1 {
              }
              frame #2 {
              }
              frame #3 {
                # "CAL;A1;<true_T>"
                n745 = local write "Due Write"("CAL;A1;60" ("Command")) -> ()
              }
              frame #4 {
                n746 = Wait (ms)(milliseconds to wait=u32 1000) -> ()  [unwired: 1 out]
              }
              frame #5 {
                # "CAL;A1;<true_T>"
                n747 = local read "Sensor value"() -> (→"Sample 60deg temp":dbl)
                n748 = local write "Due Write"("CAL;A1;60" ("Command")) -> ()
              }
            }
          }
          frame #1 {
            w793 = 0.0
            w794 = 60.0
            n749 = local read "Sample 0deg temp"() -> (w804:dbl)
            n750 = local read "Sample 60deg temp"() -> (w803:dbl)
            n751 = Add(x=w794, y="Temperature diff") -> (x+y=w801:dbl)
            n752 = Subtract(x=w794, y="Temperature diff") -> (x-y=w800:dbl)
            n753 = Add(x=w793, y="Temperature diff") -> (x+y=w799:dbl)
            n754 = Subtract(x=w793, y="Temperature diff") -> (x-y=w798:dbl)
            n755 = In Range and Coerce(upper limit=w801, x=w803, lower limit=w800) -> (In Range?=w797:bool)  [unwired: 1 out]
            n756 = In Range and Coerce(upper limit=w799, x=w804, lower limit=w798) -> (In Range?=w796:bool)  [unwired: 1 out]
            n757 = And(x=w797, y=w796) -> (x .and. y?=w795:bool)
            n758 = case shown="True" w795 {
              frame False {
                n759 = property on="Accept & Save sample Temperature step 4" class="Bool (strict)"("DisabledEnum"=T19."Disabled" ("Disabled")) -> ()  [unwired: 2 in, 2 out]
                n760 = local write "Sample Temperature Calibration"(enum32{"True", "Fail"}."Fail" ("Sample Temperature Calibration  2")) -> ()
              }
              frame True {
                n761 = property on="Accept & Save sample Temperature step 4" class="Bool (strict)"("DisabledEnum"=T19."Enabled" ("Disabled")) -> ()  [unwired: 2 in, 2 out]
                n762 = local write "Sample Temperature Calibration"(enum32{"True", "Fail"}."True" ("Sample Temperature Calibration  2")) -> ()
              }
            }
          }
          frame #2 {
          }
          frame #3 {
          }
          frame #4 {
          }
          frame #5 {
          }
          frame #6 {
            # "CAL;END"
          }
          frame #7 {
          }
          frame #8 {
            # "CAL;END"
          }
          frame #9 {
            n763 = local write "Tab Control 4"(T12."Step 4" ("Tab Control 4")) -> ()
          }
        }
      }
      event "Accept & Save sample Temperature step 4": Value Change {
        n764 = event-data() -> ()  [unwired: 1 in, 6 out]
        n765 = stacked-sequence {
          frame #0 {
            n766 = local write "Due Write"("CAL;SAVE" ("Command")) -> ()
          }
          frame #1 {
            n767 = Wait (ms)(milliseconds to wait=u32 1000) -> ()  [unwired: 1 out]
          }
          frame #2 {
            n768 = local write "Due Write"("CAL;SAVE" ("Command")) -> ()
          }
          frame #3 {
            n769 = Wait (ms)(milliseconds to wait=u32 1000) -> ()  [unwired: 1 out]
          }
          frame #4 {
            n770 = local write "Due Write"("CAL;END" ("Command")) -> ()
          }
          frame #5 {
            n771 = Wait (ms)(milliseconds to wait=u32 1000) -> ()  [unwired: 1 out]
          }
          frame #6 {
            n772 = local write "Due Write"("CAL;END" ("Command")) -> ()
            n773 = local write "Temperature Selection"(T13."Default" ("Temperature Selection")) -> ()
            n774 = local write "Calibration Selection"(T8."Default" ("Calibration Selection")) -> ()
            n775 = local write "Tab Control 4"(T12."Main" ("Tab Control 4")) -> ()
            n776 = local write "Main Calibration Tab"(T7."Temperature" ("Main Calibration Tab")) -> ()
          }
          frame #7 {
            n777 = Get Date/Time In Seconds() -> (seconds since 1Jan1904=w823:timestamp)
            n778 = Format Into String(format string="%<%I:%M:%S:%p %d:%B:%Y>T", w823) -> (resulting string=w821:string)  [unwired: 2 in, 1 out]
            n779 = local write "TEMPERATURE CALIBRATION"(w821) -> ()
          }
          frame #8 {
            n780 = local write "Save Button"(TRUE ("Save Button")) -> ()
            n781 = local write "Tab Control 4"(T12."Main" ("Tab Control 4")) -> ()
          }
        }
      }
      event "Accept & Save Air Temperature step 4": Value Change {
        n782 = event-data() -> ()  [unwired: 1 in, 6 out]
        n783 = stacked-sequence {
          frame #0 {
            n784 = local write "Due Write"("CAL;SAVE" ("Command")) -> ()
          }
          frame #1 {
            n785 = Wait (ms)(milliseconds to wait=u32 1000) -> ()  [unwired: 1 out]
          }
          frame #2 {
            n786 = local write "Due Write"("CAL;SAVE" ("Command")) -> ()
          }
          frame #3 {
            n787 = Wait (ms)(milliseconds to wait=u32 1000) -> ()  [unwired: 1 out]
          }
          frame #4 {
            n788 = local write "Due Write"("CAL;END" ("Command")) -> ()
          }
          frame #5 {
            n789 = Wait (ms)(milliseconds to wait=u32 1000) -> ()  [unwired: 1 out]
          }
          frame #6 {
            n790 = local write "Due Write"("CAL;END" ("Command")) -> ()
            n791 = local write "Tab Control 4"(T12."Main" ("Tab Control 4")) -> ()
            n792 = local write "Main Calibration Tab"(T7."Temperature" ("Main Calibration Tab")) -> ()
            n793 = local write "Temperature Selection"(T13."Default" ("Temperature Selection")) -> ()
            n794 = local write "Calibration Selection"(T8."Default" ("Calibration Selection")) -> ()
          }
          frame #7 {
            n795 = Get Date/Time In Seconds() -> (seconds since 1Jan1904=w839:timestamp)
            n796 = Format Into String(format string="%<%I:%M:%S:%p %d:%B:%Y>T", w839) -> (resulting string=w838:string)  [unwired: 2 in, 1 out]
            n797 = local write "TEMPERATURE CALIBRATION"(w838) -> ()
          }
          frame #8 {
            n798 = local write "Tab Control 4"(T12."Main" ("Tab Control 4")) -> ()
            n799 = local write "Save Button"(TRUE ("Save Button")) -> ()
          }
        }
      }
      event "Temperature Continue Step 6": Value Change {
        n800 = event-data() -> ()  [unwired: 1 in, 6 out]
        n801 = stacked-sequence {
          frame #0 {
            n802 = stacked-sequence {
              frame #0 {
                n803 = Wait (ms)(milliseconds to wait=u32 1000) -> ()  [unwired: 1 out]
              }
              frame #1 {
              }
              frame #2 {
              }
              frame #3 {
                # "CAL;A1;<true_T>"
                n804 = local write "Due Write"("CAL;A1;60" ("Command")) -> ()
              }
              frame #4 {
                n805 = Wait (ms)(milliseconds to wait=u32 1000) -> ()  [unwired: 1 out]
              }
              frame #5 {
                # "CAL;A1;<true_T>"
                n806 = local write "Due Write"("CAL;A1;60" ("Command")) -> ()
              }
            }
          }
          frame #1 {
            n807 = local read "Sensor value"() -> (→"Air 60deg temp":dbl)
          }
          frame #2 {
          }
          frame #3 {
          }
          frame #4 {
          }
          frame #5 {
          }
          frame #6 {
            # "CAL;END"
          }
          frame #7 {
            w847 = 0.0 ("x")
            w848 = 60.0 ("x")
            n808 = local read "Temperature diff"() -> (w851:dbl)
            n809 = local read "Air 60deg temp"() -> (w850:dbl)
            n810 = local read "Air 0deg temp"() -> (w849:dbl)
            n811 = Add(x=w848, y=w851) -> (x+y=w858:dbl)
            n812 = Subtract(x=w848, y=w851) -> (x-y=w857:dbl)
            n813 = Add(x=w847, y=w851) -> (x+y=w856:dbl)